vi "Feedback 適應性控制 NLMS(雜訊消除).vi"() -> ()   [LabVIEW 2010]
uses:
  <vilib>/DAQmx/read.llb/DAQmx Read (Analog 1D DBL NChan 1Samp).vi
  <vilib>/DAQmx/write.llb/DAQmx Write (Analog DBL 1Chan 1Samp).vi
  <vilib>/DAQmx/create/channels.llb/DAQmx Create Channel (AI-Voltage-Basic).vi
  <vilib>/DAQmx/configure/timing.llb/DAQmx Timing (Sample Clock).vi
  <vilib>/DAQmx/create/channels.llb/DAQmx Create Channel (AO-Voltage-Basic).vi
  <vilib>/daqmx/miscellaneous.llb/DAQmx Fill In Error Info.vi
panel:
  out "data out":dbl[][](graph)
  out "Crest factor (peak/rms)":dbl=4.48166370874089
  out "絕對誤差 RMS":dbl=0.014061833175896706
  in  "絕對誤差Peak RMS開始計算時間(s)":dbl=10.0
  out "絕對誤差 max":dbl=0.06302040742278492
  out "均方誤差,MSE":waveform(dbl)(graph)={"t0"=timestamp(0 s since 1904-01-01), "dt"=0.0001, "Y"=array[200000 elements]}
  out "絕對平均誤差,MAE":waveform(dbl)(graph)={"t0"=timestamp(0 s since 1904-01-01), "dt"=0.0001, "Y"=array[200000 elements]}
  in  "Mode":bool=TRUE
  in  "stop time (s)":dbl=20.0
  out "絕對誤差,AE":waveform(dbl)(graph)={"t0"=timestamp(0 s since 1904-01-01), "dt"=0.0001, "Y"=array[200000 elements]}
  out "signal+noise":dbl[][](graph)=[[-0.42316279029509396, -0.4166253949171763, -0.4101340929315377], [-0.42316279029509396, -0.4166253949171763, -0.4101340929315377], [-0.42316279029509396, -0.4166253949171763, -0.4101340929315377]]
  in  "NLMS-r(防止過大步長)":dbl=1.0
  in  "u(收斂係數)":dbl=0.0003
  in  "order":i32=10
  in  "AO on":bool=TRUE
  out "error out":errorcluster
  out "延遲百分比(%)  需小於0.5%":dbl=0.023842294062181857
  out "理想迴圈時間(ms)":dbl=0.1
  out "迴圈平均運行時間(ms)":dbl=0.10002384229406218
  in  "output channels 1":tag="PXI-6733/ao0"
  in  "每通道取樣頻率(Hz)":dbl=10000.0 format="%0.2f"
  in  "input channels 2 (noise)":tag="PXI-6229/ai1"
  in  "input channels 1 (signal)":tag="PXI-6229/ai0"
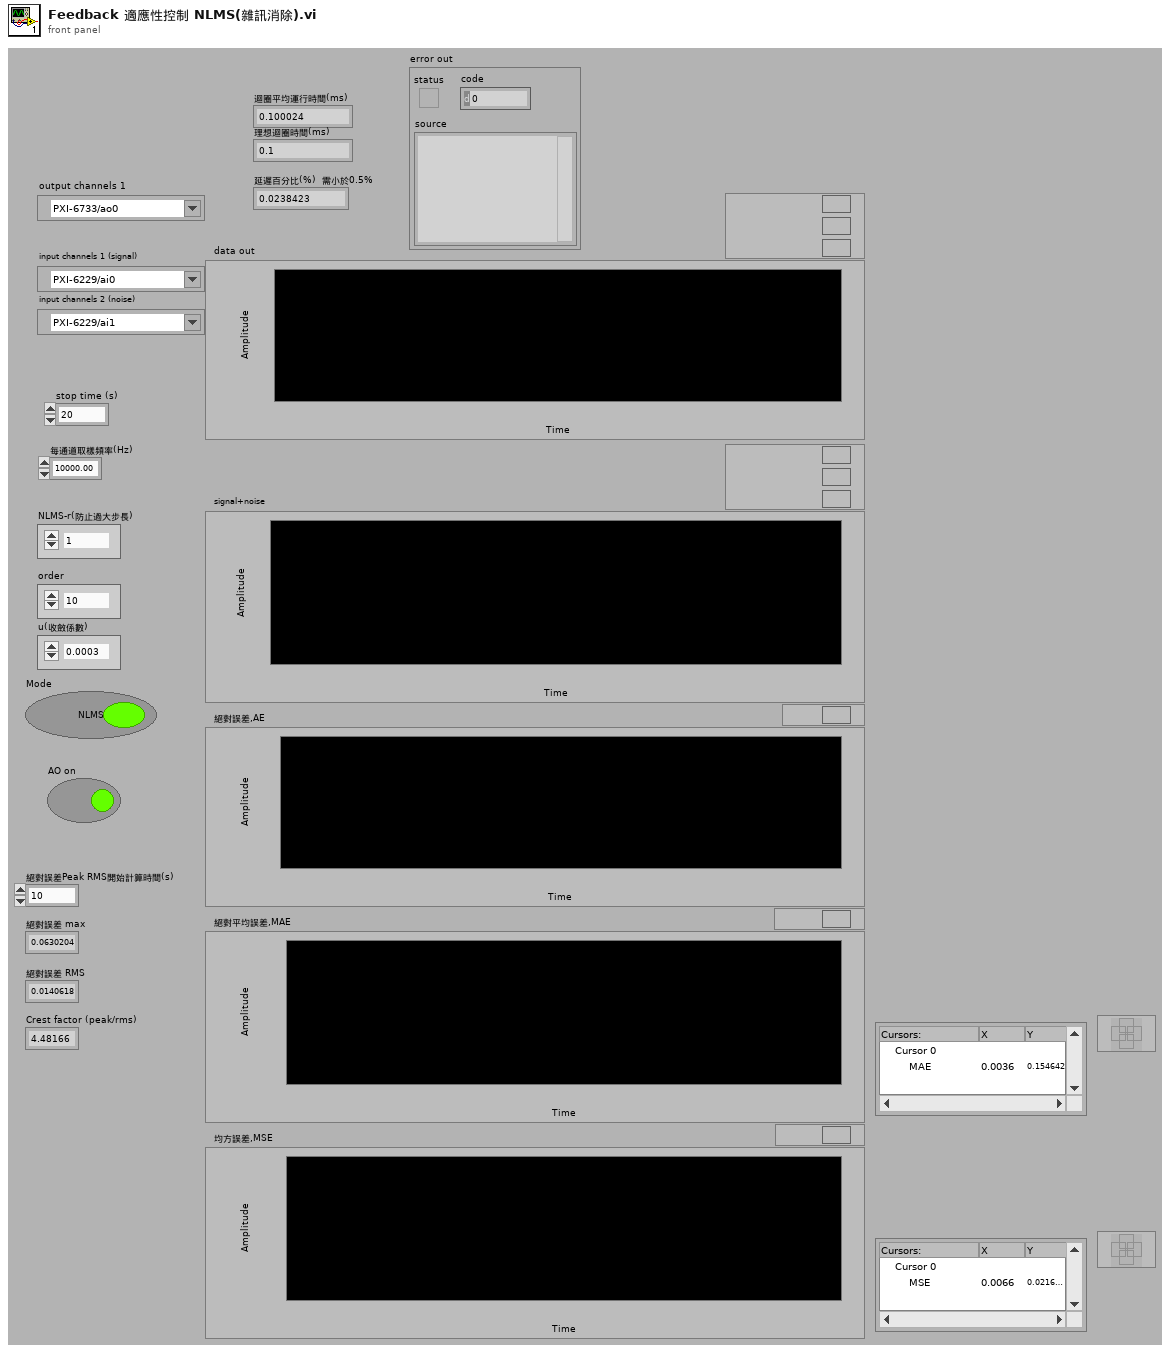
[diagram p1: front panel]
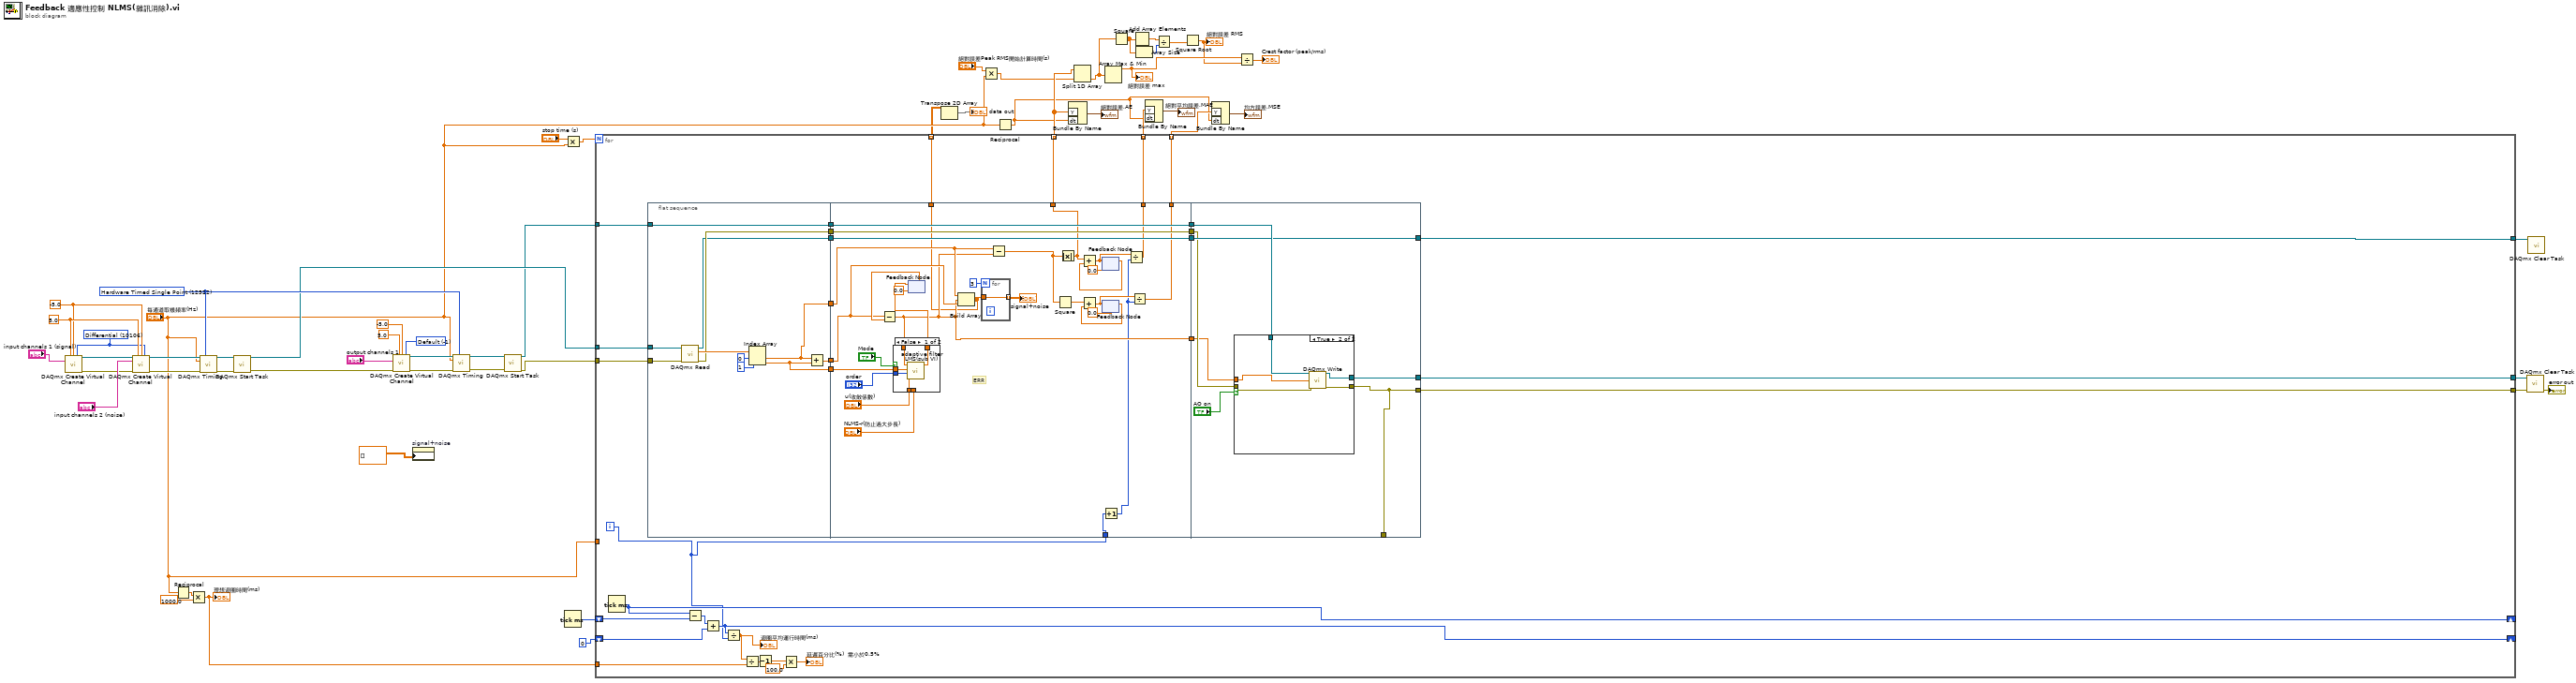
[diagram p0: block diagram]
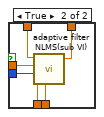
[diagram p2: hidden frame]
diagram:
  w43 = -1 items=["Default"=-1, "RSE"=10083, "Differential"=10106, "Pseudodifferential"=12529] ("output terminal configuration")
  w40 = 12522 items=["Finite Samples"=10178, "Continuous Samples"=10123, "Hardware Timed Single Point"=12522] ("sample mode")
  w51 = 10106 items=["default"=-1, "RSE"=10083, "NRSE"=10078, "Differential"=10106, "Pseudodifferential"=12529] ("input terminal configuration")
  w52 = -5.0 ("minimum value")
  w53 = 5.0 ("maximum value")
  n1 = call-poly <vilib>:"DAQmx Create Virtual Channel.vi"("maximum value"=w53, "minimum value"=w52, "input terminal configuration"=w51, "physical channels"="input channels 1 (signal)") -> ("task out"=w56:refnum<k21>, "error out"=w48:errorcluster)  [unwired: 10 in]
  n2 = call-poly <vilib>:"DAQmx Create Virtual Channel.vi"("task in"=w56, "maximum value"=w53, "minimum value"=w52, "input terminal configuration"=w51, "physical channels"="input channels 2 (noise)", "error in"=w48) -> ("task out"=w50:refnum<k21>, "error out"=w47:errorcluster)  [unwired: 8 in]
  n3 = Reciprocal(x="每通道取樣頻率(Hz)") -> (1/x=w31:dbl)
  n4 = Multiply(x=w31, y=1000.0) -> (x*y=w29:dbl)
  "理想迴圈時間(ms)" <- w29
  n5 = call-poly <vilib>:"DAQmx Timing.vi"("task/channels in"=w50, "sample mode"=w40, "rate"="每通道取樣頻率(Hz)", "error in"=w47) -> ("task out"=w49:refnum<k21>, "error out"=w46:errorcluster)  [unwired: 10 in]
  n6 = call <vilib>:"DAQmx Start Task.vi"("task/channels in"=w49, "error in"=w46) -> ("task out"=w36:refnum<k21>, "error out"=w37:errorcluster)  [unwired: 12 in]
  n7 = call-poly <vilib>:"DAQmx Create Virtual Channel.vi"("maximum value"=5.0, "minimum value"=-5.0 ("maximum value"), "output terminal configuration"=w43, "physical channels"="output channels 1", "error in"=w37) -> ("task out"=w42:refnum<k21>, "error out"=w41:errorcluster)  [unwired: 9 in]
  n8 = property on="signal+noise" class="WFChart (strict)"("History Data"=dbl[][] []) -> ()  [unwired: 2 in, 2 out]
  n9 = call-poly <vilib>:"DAQmx Timing.vi"("task/channels in"=w42, "sample mode"=w40, "rate"="每通道取樣頻率(Hz)", "error in"=w41) -> ("task out"=w39:refnum<k21>, "error out"=w38:errorcluster)  [unwired: 10 in]
  n10 = call <vilib>:"DAQmx Start Task.vi"("task/channels in"=w39, "error in"=w38) -> ("task out"=w28:refnum<k21>, "error out"=w35:errorcluster)  [unwired: 12 in]
  n11 = Tick Count (ms)() -> (millisecond timer value=w33:u32)
  n12 = Multiply(x="stop time (s)", y="每通道取樣頻率(Hz)") -> (x*y=w21:dbl)
  n13 = for {
    N: w21 -> [_]
    tunnel: w36 -> [w88]
    tunnel: w35 -> [w87]
    shift-right: [w63] -> _
    shift-left: w33 -> [w86]
    shift-right: [w83] -> _
    shift-left: 0 ("index") -> [w84]
    tunnel: w29 -> [w81]
    tunnel: "每通道取樣頻率(Hz)" -> [_]
    tunnel: w28 -> [w76]
    tunnel: [w75] -> w26
    tunnel: [w73] -> w25
    tunnel: [w74] -> w24
    tunnel: [w61] -> w15 mode=indexing
    tunnel: [w59] -> w18 mode=indexing
    tunnel: [w58] -> w16 mode=indexing
    tunnel: [w57] -> w2 mode=indexing
    i -> [w60]
    n14 = Tick Count (ms)() -> (millisecond timer value=w63:u32)
    n15 = flat-sequence {
      tunnel: w88 -> [w99]
      tunnel: w87 -> [w98]
      tunnel: w76 -> [w94]
      tunnel: [w94] -> w69
      tunnel: [w93] -> w68
      tunnel: [w92] -> w67
      tunnel: [w91] -> w66
      tunnel: [w89] -> w65
      tunnel: [w90] -> w62
      tunnel: w69 -> [w129]
      tunnel: [w129] -> w72
      tunnel: w68 -> [w128]
      tunnel: [w128] -> w71
      tunnel: w67 -> [w127]
      tunnel: [w127] -> w70
      tunnel: w66 -> [w118]
      tunnel: w65 -> [w114]
      tunnel: [w116] -> w64
      tunnel: w62 -> [w117]
      tunnel: [w101] -> w61
      tunnel: w60 -> [w110]
      tunnel: [w109] -> w59
      tunnel: [w102] -> w58
      tunnel: [w100] -> w57
      tunnel: w72 -> [w148]
      tunnel: [w147] -> w75
      tunnel: w71 -> [w144]
      tunnel: [w143] -> w73
      tunnel: [w146] -> w74
      tunnel: w70 -> [w146]
      tunnel: [w143] -> _
      tunnel: w64 -> [w142]
      frame #0 {
        n16 = call-poly <vilib>:"DAQmx Read.vi"("task/channels in"=w99, "error in"=w98) -> ("task out"=w92:refnum<k21>, "data"=w95:dbl[], "error out"=w93:errorcluster)  [unwired: 11 in]
        n17 = Index Array(array=w95, index #1=0 ("index"), index #2=1 ("index")) -> (element #1=w90:dbl, element #2=w89:dbl)
        n18 = Add(x=w90, y=w89) -> (x+y=w91:dbl)
      }
      frame #1 {
        # "ERR"
        n19 = feedback #1(0.0 ("FIR輸出")) -> (w123:dbl)
        n20 = Subtract(x=w118, y=w123) -> (x-y=w116:dbl)
        n21 = case shown="False" "Mode" {
          tunnel: "order" -> [w131 w140]
          tunnel: "u(收斂係數)" -> [w130 w139]
          tunnel: [w133 w138] -> w124
          tunnel: "NLMS-r(防止過大步長)" -> [_ w137]
          tunnel: w114 -> [w132 w136]
          tunnel: w116 -> [w134 w135]
          frame False {
            n22 = call "adaptive filter LMS(sub VI).vi"("ERR"=w134, "輸入訊號"=w132, "order"=w131, "u(收斂係數)"=w130) -> ("FIR輸出"=w133:dbl)  [unwired: 3 in, 1 out]
          }
          frame True {
            n23 = call "adaptive filter NLMS(sub VI).vi"("ERR"=w135, "NLMS-r(防止過大步長)"=w137, "輸入訊號"=w136, "order"=w140, "u(收斂係數)"=w139) -> ("FIR輸出"=w138:dbl)  [unwired: 2 in, 1 out]
          }
        }
        n24 = feedback-in #1(w124) -> ()
        n25 = Build Array(w117, w116, w118) -> (w100:dbl[])
        n26 = for {
          N: 3 -> [_]
          tunnel: w100 -> [w141]
          tunnel: [w141] -> w120 mode=indexing
        }
        "signal+noise" <- w120
        n27 = Subtract(x=w117, y=w116) -> (x-y=w108:dbl)
        n28 = Square(x=w108) -> (x^2=w106:dbl)
        n29 = Absolute Value(x=w108) -> (abs(x)=w101:dbl)
        n30 = feedback #2(0.0) -> (w113:dbl)
        n31 = Add(x=w101, y=w113) -> (x+y=w111:dbl)
        n32 = feedback-in #2(w111) -> ()
        n33 = feedback #3(0.0) -> (w105:dbl)
        n34 = Add(x=w106, y=w105) -> (x+y=w104:dbl)
        n35 = feedback-in #3(w104) -> ()
        n36 = Increment(x=w110) -> (x+1=w103:i32)
        n37 = Divide(x=w111, y=w103) -> (x/y=w109:dbl)
        n38 = Divide(x=w104, y=w103) -> (x/y=w102:dbl)
      }
      frame #2 {
        n39 = case shown="True" "AO on" {
          tunnel: w148 -> [_ w153]
          tunnel: [_ w152] -> w147
          tunnel: w144 -> [_ w151]
          tunnel: [_ w150] -> w143
          tunnel: w142 -> [_ w149]
          frame False {
          }
          frame True {
            n40 = call-poly <vilib>:"DAQmx Write.vi"("task/channels in"=w153, "data"=w149, "error in"=w151) -> ("task out"=w152:refnum<k21>, "error out"=w150:errorcluster)  [unwired: 10 in, 1 out]
          }
        }
      }
    }
    n41 = Subtract(x=w63, y=w86) -> (x-y=w85:u32)
    n42 = Add(x=w85, y=w84) -> (x+y=w83:u32)
    n43 = Divide(x=w83, y=w60) -> (x/y=w82:dbl)
    "迴圈平均運行時間(ms)" <- w82
    n44 = Divide(x=w82, y=w81) -> (x/y=w80:dbl)
    n45 = Decrement(x=w80) -> (x-1=w79:dbl)
    n46 = Multiply(x=w79, y=100.0) -> (x*y=→"延遲百分比(%)  需小於0.5%":dbl)
  }
  n47 = Transpose 2D Array(2D array=w2) -> (transposed array=→"data out":dbl[][])
  n48 = Multiply(x="絕對誤差Peak RMS開始計算時間(s)", y="每通道取樣頻率(Hz)") -> (x*y=w13:dbl)
  n49 = Reciprocal(x="每通道取樣頻率(Hz)") -> (1/x=w3:dbl)
  n50 = Bundle By Name("Y"=w15, "dt"=w3) -> (→"絕對誤差,AE":waveform(dbl))  [unwired: 1 in]
  n51 = Split 1D Array(array=w15, index=w13) -> (second subarray=w11:dbl[])  [unwired: 1 out]
  n52 = Array Max & Min(array=w11) -> (max value=w6:dbl)  [unwired: 3 out]
  "絕對誤差 max" <- w6
  n53 = Square(x=w11) -> (x^2=w8:dbl[])
  n54 = Add Array Elements(numeric array=w8) -> (sum=w10:dbl)
  n55 = Array Size(array=w8) -> (size(s)=w9:i32)
  n56 = Bundle By Name("Y"=w18, "dt"=w3) -> (→"絕對平均誤差,MAE":waveform(dbl))  [unwired: 1 in]
  n57 = Divide(x=w10, y=w9) -> (x/y=w7:dbl)
  n58 = Square Root(x=w7) -> (sqrt(x)=w5:dbl)
  "絕對誤差 RMS" <- w5
  n59 = Bundle By Name("Y"=w16, "dt"=w3) -> (→"均方誤差,MSE":waveform(dbl))  [unwired: 1 in]
  n60 = Divide(x=w6, y=w5) -> (x/y=→"Crest factor (peak/rms)":dbl)
  n61 = call <vilib>:"DAQmx Clear Task.vi"("task in"=w26, "error in"=w25) -> ("error out"=→"error out":errorcluster)  [unwired: 13 in]
  n62 = call <vilib>:"DAQmx Clear Task.vi"("task in"=w24) -> ()  [unwired: 14 in, 1 out]
